vi "Main Test.vi"() -> ()   [LabVIEW 2020]
uses:
  Mete.ctl
  R.ctl
  P.ctl
  N.ctl
  D.ctl
  Odo Velocity.ctl
  Gas.ctl
  Set-.ctl
  Set+.ctl
  Cru.ctl
  Dis.ctl
  CharRPM.ctl
  CharODO.ctl
  Brake.ctl
  Limit.ctl
panel:
  in  "Limit":T1
  out "Image":T2(plugin-control)
  in  "Slide 4":T3 scale=0.0..700.0
  in  "Slide 3":dbl(slide) scale=0.0..10.0
  out "Waveform Chart":T4
  out "Waveform Chart 2":T5
  in  "Dis":T6 caption="Boolean 8"
  in  "Cu":T7 caption="Boolean 7"
  in  "+Cu":T8 caption="Boolean 5"
  in  "-Cu":T9 caption="Boolean 6"
  in  "Slide 2":T10 scale=0.0..700.0
  out "Km/h":T11 scale=0.0..250.0
  in  "stop":bool
  in  "Slide":u32(slide) max=300 scale=0.0..650.0
  out "Boolean 4":T12
  out "Boolean 3":T13
  out "Boolean 2":T14
  out "Boolean":T15
  out "Gauge":T16 scale=0.0..650.0
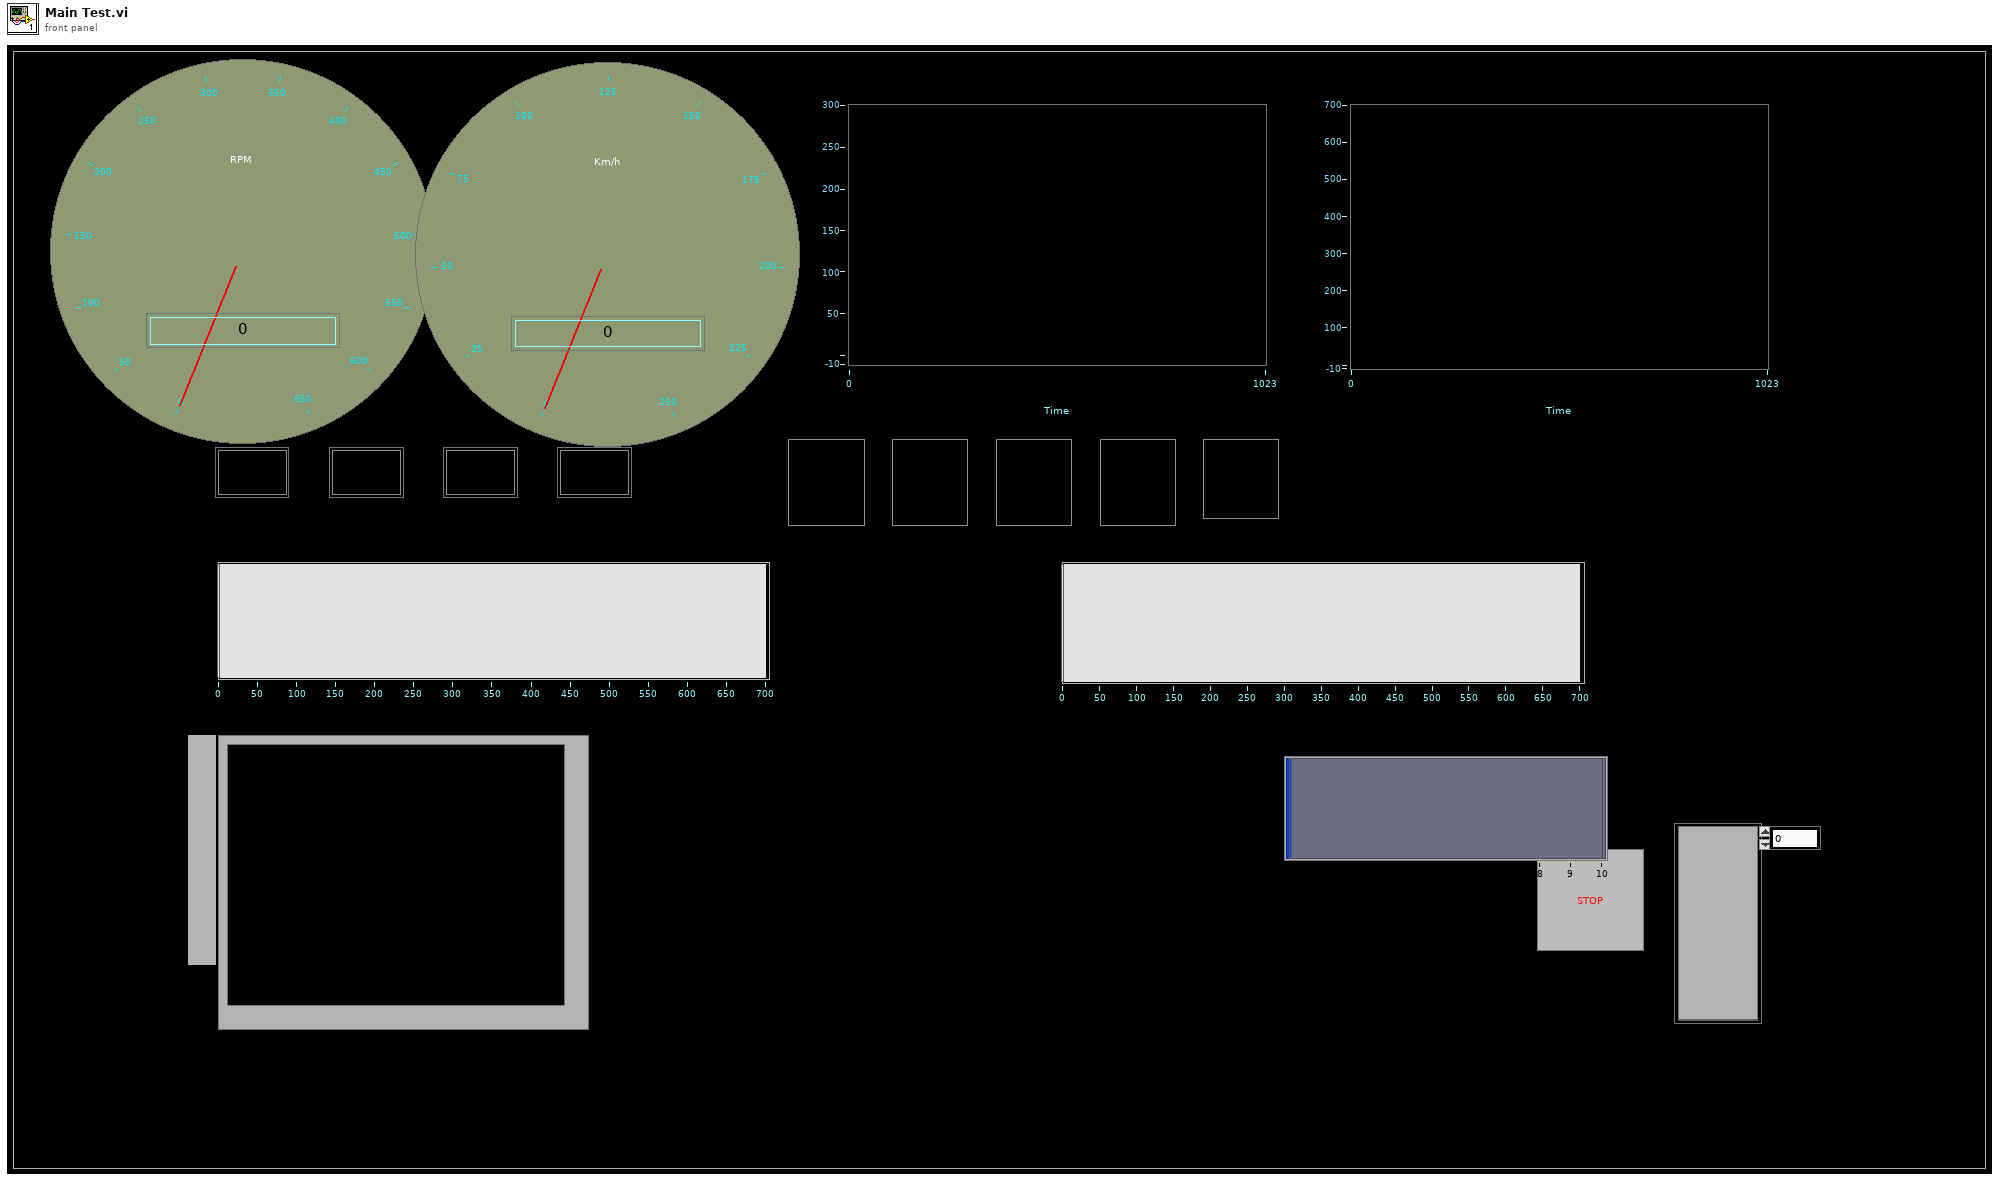
[diagram p1: front panel]
types:
  T1 = typedef "Limit.ctl" = bool
  T2 = typedef "IMAQ Image.ctl" = refnum<image>
  T3 = typedef "Brake.ctl" = dbl
  T4 = typedef "CharODO.ctl" = dbl
  T5 = typedef "CharRPM.ctl" = dbl
  T6 = typedef "Dis.ctl" = bool
  T7 = typedef "Cru.ctl" = bool
  T8 = typedef "Set+.ctl" = bool
  T9 = typedef "Set-.ctl" = bool
  T10 = typedef "Gas.ctl" = dbl
  T11 = typedef "Odo Velocity.ctl" = u16
  T12 = typedef "D.ctl" = bool
  T13 = typedef "N.ctl" = bool
  T14 = typedef "P.ctl" = bool
  T15 = typedef "R.ctl" = bool
  T16 = typedef "Mete.ctl" = u16
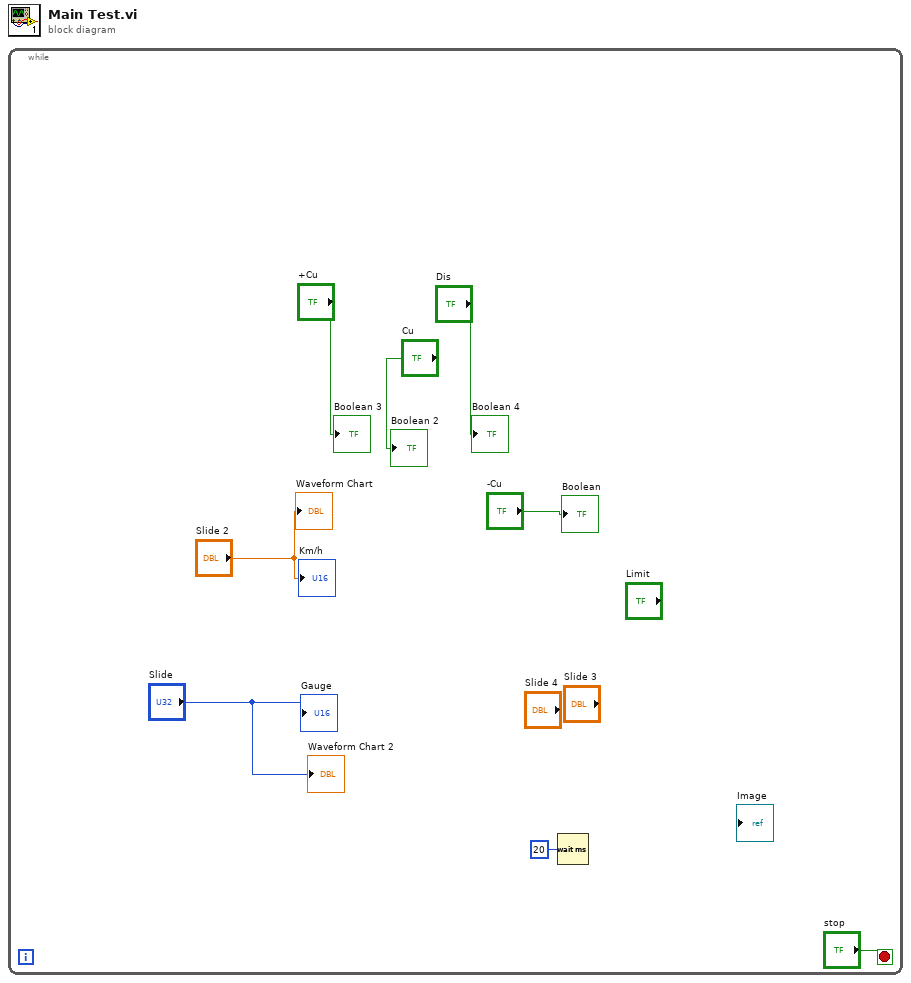
[diagram p0: block diagram]
diagram:
  n1 = while {
    stop <- "stop" stop-if-true
    n2 = Wait (ms)(milliseconds to wait=u32 20) -> ()  [unwired: 1 out]
    "Gauge" <- "Slide"
    "Boolean 2" <- "Cu"
    "Boolean 3" <- "+Cu"
    "Boolean" <- "-Cu"
    "Boolean 4" <- "Dis"
    "Km/h" <- "Slide 2"
    "Waveform Chart 2" <- "Slide"
    "Waveform Chart" <- "Slide 2"
  }
